vi "Grab -Main-CCD1 - 2.vi"(0 "Image in":T6(plugin-control)=refnum, 2 "right":dbl=1152.0, 3 "left":dbl=846.0, 5 "显示抓取图像":bool=TRUE, 7 "CCD2参数":T5={"Rectangle"={"Left"=1952, "Top"=146, "Right"=370, "Bottom"=2690, "Rotation"=45.0}, "Angle (degrees) "=90.0, "long"=150.0, "abgek"=-90.0, "Color"=16711680, "left threshold"=0.0, "Rectangle right"={"Left"=1952, "Top"=1596, "Right"=570, "Bottom"=2690, "Rotation"=45.0}, "long right"=150.0, "abgek right"=90.0, "Color 2"=16711680, "right threshold"=0.0, "left"=0.0, "right"=0.0, "Settings (Big)"={"Extraction Mode"=0, "Edge Threshold"=17, "Edge Filter Size"=1, "Min Length"=36, "Row Search Step Size"=13, "Col Search Step Size"=13, "Max Endpoint Gap"=10, "Closed"=FALSE, "Subpixel"=TRUE}, "Clamp Settings (Big)"={"Angle "=10.0, "Edge Polarity"={"Start"=0, "End"=0}}, " Settings top"={"Extraction Mode"=0, "Edge Threshold"=18, "Edge Filter Size"=1, "Min Length"=36, "Row Search Step Size"=64, "Col Search Step Size"=64, "Max Endpoint Gap"=10, "Closed"=FALSE, "Subpixel"=TRUE}, "Clamp Settings top "={"Angle "=10.0, "Edge Polarity"={"Start"=0, "End"=0}}, "Sub-Pixel Accuracy "=TRUE, "Threshold Parameters"={"Level Type"=enum."Absolute Value", "Threshold Level"=127, "Hysteresis"=2}, "Process "=enum."Get First + Last Edge", "Threshold Parameters 2"={"Level Type"=enum."Absolute Value", "Threshold Level"=127, "Hysteresis"=2}} {"Clamp Settings top"."Edge Polarity"."Start" items=["Any", "Rising", "Falling"]; "Clamp Settings top"."Edge Polarity"."End" items=["Any", "Rising", "Falling"]; "Settings top"."Extraction Mode" items=["Normal", "Uniform Regions"]; "Settings top"."Edge Filter Size" items=["Fine", "Normal", "Contour Tracing"]; "Settings top"."Max Endpoint Gap" min=0; "Settings top"."Col Search Step Size" min=1 max=255 step=1; "Settings top"."Row Search Step Size" min=1 max=255 step=1; "Settings top"."Min Length" min=0; "Settings top"."Edge Threshold" min=1 max=350 step=1; "Clamp Settings (Big)"."Edge Polarity"."Start" items=["Any", "Rising", "Falling"]; "Clamp Settings (Big)"."Edge Polarity"."End" items=["Any", "Rising", "Falling"]; "Settings (Big)"."Extraction Mode" items=["Normal", "Uniform Regions"]; "Settings (Big)"."Edge Filter Size" items=["Fine", "Normal", "Contour Tracing"]; "Settings (Big)"."Max Endpoint Gap" min=0; "Settings (Big)"."Col Search Step Size" min=1 max=255 step=1; "Settings (Big)"."Row Search Step Size" min=1 max=255 step=1; "Settings (Big)"."Min Length" min=0; "Settings (Big)"."Edge Threshold" min=1 max=350 step=1; "Rectangle right"."Rotation" format="%.2f"; "Rectangle right"."Left" scale=0.0..1024.0; "Rectangle right"."Right" scale=0.0..1024.0; "Rectangle"."Rotation" format="%.2f"; "Rectangle"."Left" scale=0.0..1024.0; "Rectangle"."Right" scale=0.0..1024.0}, 9 "ROI参数":T3={"Rectangle big CCD1"={"Left"=1952, "Top"=1596, "Right"=570, "Bottom"=2690, "Rotation"=45.0}, "Rectangle top CCD1 "={"Left"=1952, "Top"=1596, "Right"=570, "Bottom"=2690, "Rotation"=45.0}, "Line"={"Start X"=0, "Start Y"=0, "End X"=0, "End Y"=0}, "left line "=846.0, "right line"=1152.0} {"Line"."Start X" scale=0.0..1024.0; "Line"."End X" scale=0.0..1024.0; "Rectangle top CCD1"."Rotation" format="%.2f"; "Rectangle top CCD1"."Left" scale=0.0..1024.0; "Rectangle top CCD1"."Right" scale=0.0..1024.0; "Rectangle big CCD1"."Rotation" format="%.2f"; "Rectangle big CCD1"."Left" scale=0.0..1024.0; "Rectangle big CCD1"."Right" scale=0.0..1024.0}, 11 "error in (no error)":errorcluster caption="错误输入（无错误）") -> (4 "Image out":T6(plugin-control), 6 "NO LINES":bool, 8 "CCD2-L":bool, 10 "CCD2-R":bool, 15 "error out":errorcluster caption="错误输出")   [LabVIEW 2017]
doc: "The Grab VI acquires images continuously and displays the images in an image control using high-level acquisition VIs. A grab is appropriate for high-speed applications in which you need to process only one image at a time."
uses:
  <vilib>/vision/Pattern Matching.llb/IMAQ Curve Parameters.ctl
  Global System.vi
panel:
  out "下":dbl
  out "上":dbl
  in  "组合框":string(combo)="模式1"
  # "箭头指示参数"
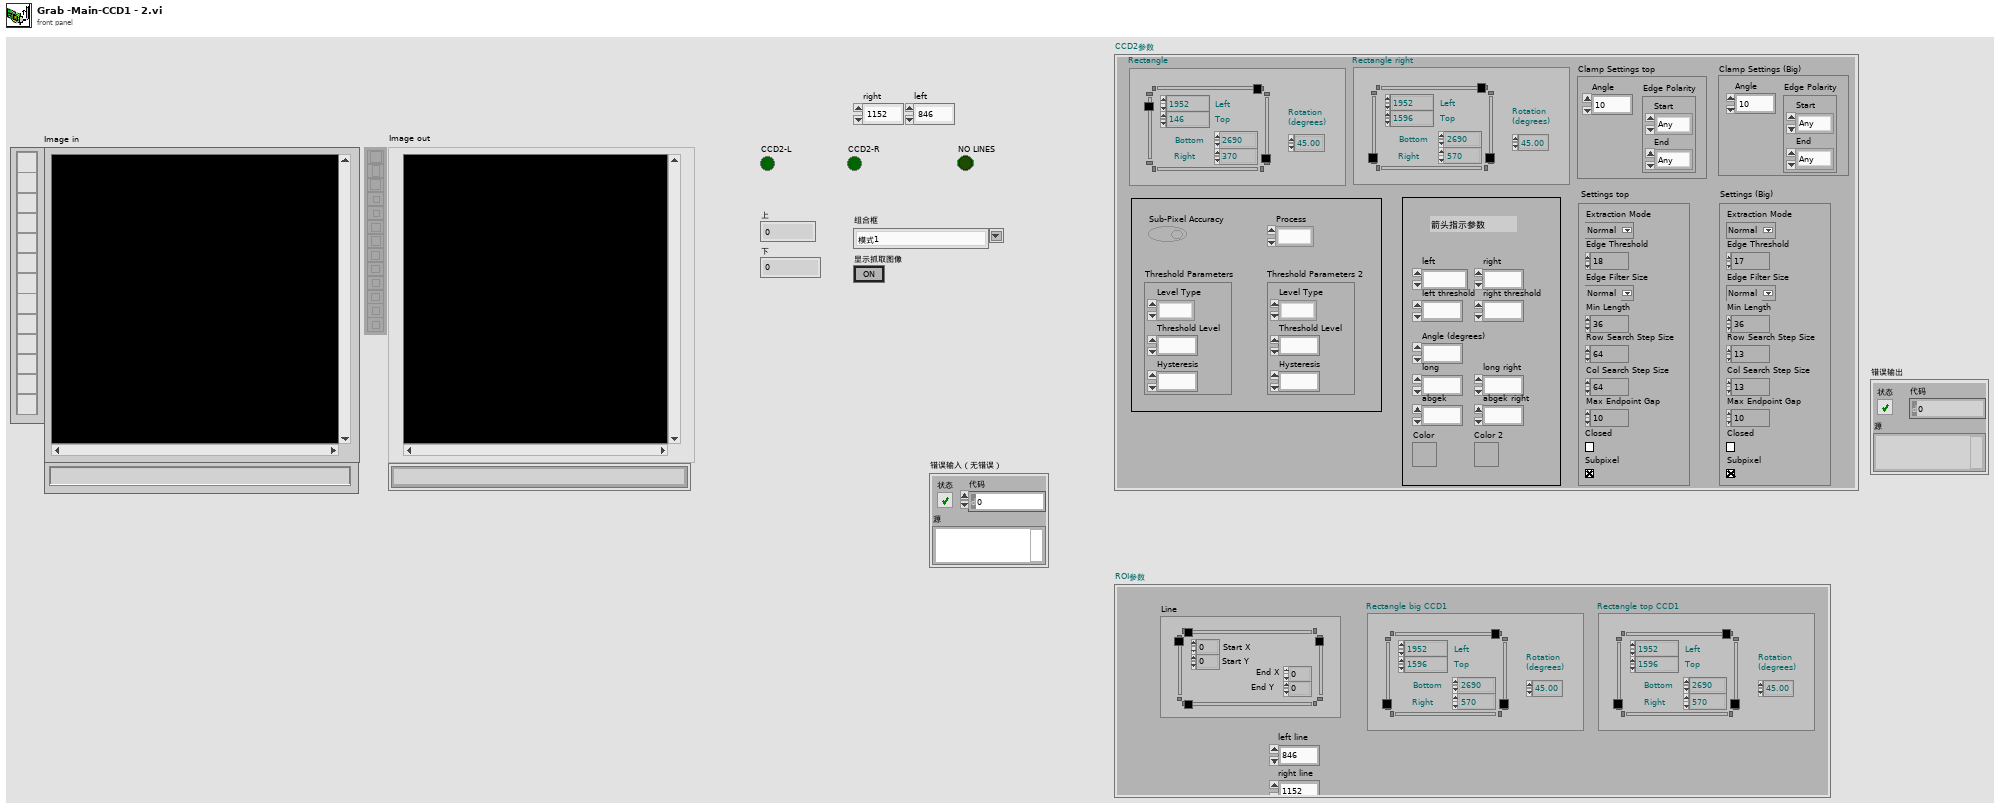
[diagram p1: front panel]
types:
  T1 = typedef "IMAQ Rectangle" = cluster{"Left":i32, "Top":i32, "Right":i32, "Bottom":i32, "Rotation":dbl}
  T2 = typedef "IMAQ Line" = cluster{"Start X":i32, "Start Y":i32, "End X":i32, "End Y":i32}
  T3 = cluster{"Rectangle big CCD1":T1, "Rectangle top CCD1 ":T1, "Line":T2, "left line ":dbl, "right line":dbl}
  T4 = typedef "IMAQ Curve Parameters.ctl" = cluster{"Extraction Mode":u32, "Edge Threshold":i32, "Edge Filter Size":u32, "Min Length":i32, "Row Search Step Size":i32, "Col Search Step Size":i32, "Max Endpoint Gap":i32, "Closed":bool, "Subpixel":bool}
  T5 = cluster{"Rectangle":T1, "Angle (degrees) ":sgl, "long":sgl, "abgek":dbl, "Color":u32, "left threshold":dbl, "Rectangle right":T1, "long right":sgl, "abgek right":dbl, "Color 2":u32, "right threshold":dbl, "left":dbl, "right":dbl, "Settings (Big)":T4, "Clamp Settings (Big)":cluster{"Angle ":dbl, "Edge Polarity":cluster{"Start":u32, "End":u32}}, " Settings top":T4, "Clamp Settings top ":cluster{"Angle ":dbl, "Edge Polarity":cluster{"Start":u32, "End":u32}}, "Sub-Pixel Accuracy ":bool, "Threshold Parameters":cluster{"Level Type":enum32{"Absolute Value", "Relative value"}, "Threshold Level":i32, "Hysteresis":i32}, "Process ":enum16{"Get First Edge", "Get First + Last Edge", "Get All Edges"}, "Threshold Parameters 2":cluster{"Level Type":enum32{"Absolute Value", "Relative value"}, "Threshold Level":i32, "Hysteresis":i32}}
  T6 = typedef "IMAQ Image.ctl" = refnum<image>
  T7 = cluster{"Clamp Points (Max Clamp 1)":cluster{"Pixels ":cluster{"Start":cluster{"X":dbl, "Y":dbl}, "End":cluster{"X":dbl, "Y":dbl}}, "Real World":cluster{"Start":cluster{"X":dbl, "Y":dbl}, "End":cluster{"X":dbl, "Y":dbl}}}, "Clamp Points (Max Clamp 2)":cluster{"Pixels ":cluster{"Start":cluster{"X":dbl, "Y":dbl}, "End":cluster{"X":dbl, "Y":dbl}}, "Real World":cluster{"Start":cluster{"X":dbl, "Y":dbl}, "End":cluster{"X":dbl, "Y":dbl}}}, "Clamp Points(top)":cluster{"Pixels ":cluster{"Start":cluster{"X":dbl, "Y":dbl}, "End":cluster{"X":dbl, "Y":dbl}}, "Real World":cluster{"Start":cluster{"X":dbl, "Y":dbl}, "End":cluster{"X":dbl, "Y":dbl}}}}
  T8 = cluster{"Angle ":dbl, "Edge Polarity":cluster{"Start":u32, "End":u32}}
  T9 = cluster{"Global Rectangle":i32[], "Contours":cluster{"ID":enum32{"External", "Internal"}, "Type":u32, "Coordinates":i32[]}[]}
  T10 = cluster{"Start":cluster{"X":dbl, "Y":dbl}, "End":cluster{"X":dbl, "Y":dbl}}
  T11 = cluster{"Pixels ":cluster{"Start":cluster{"X":dbl, "Y":dbl}, "End":cluster{"X":dbl, "Y":dbl}}, "Real World":cluster{"Start":cluster{"X":dbl, "Y":dbl}, "End":cluster{"X":dbl, "Y":dbl}}}
  T12 = cluster{"Left":i32, "Top":i32, "Right":i32, "Bottom":i32}
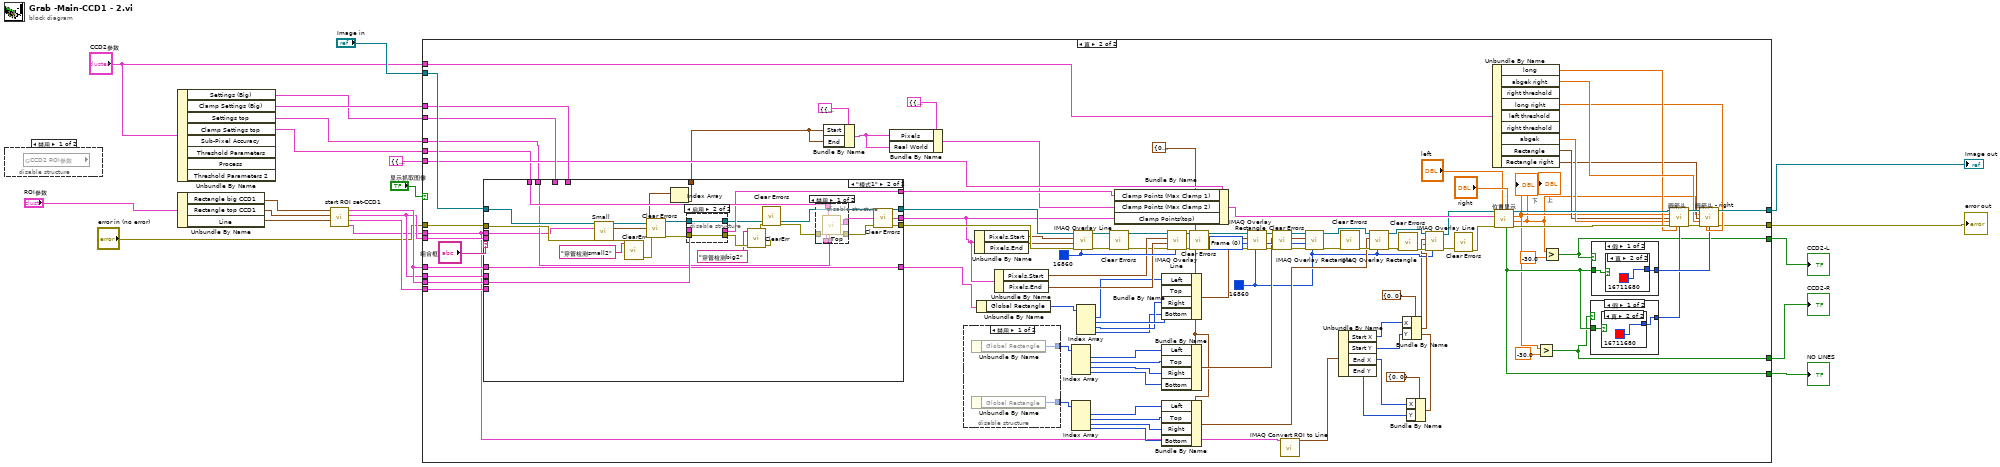
[diagram p0: block diagram]
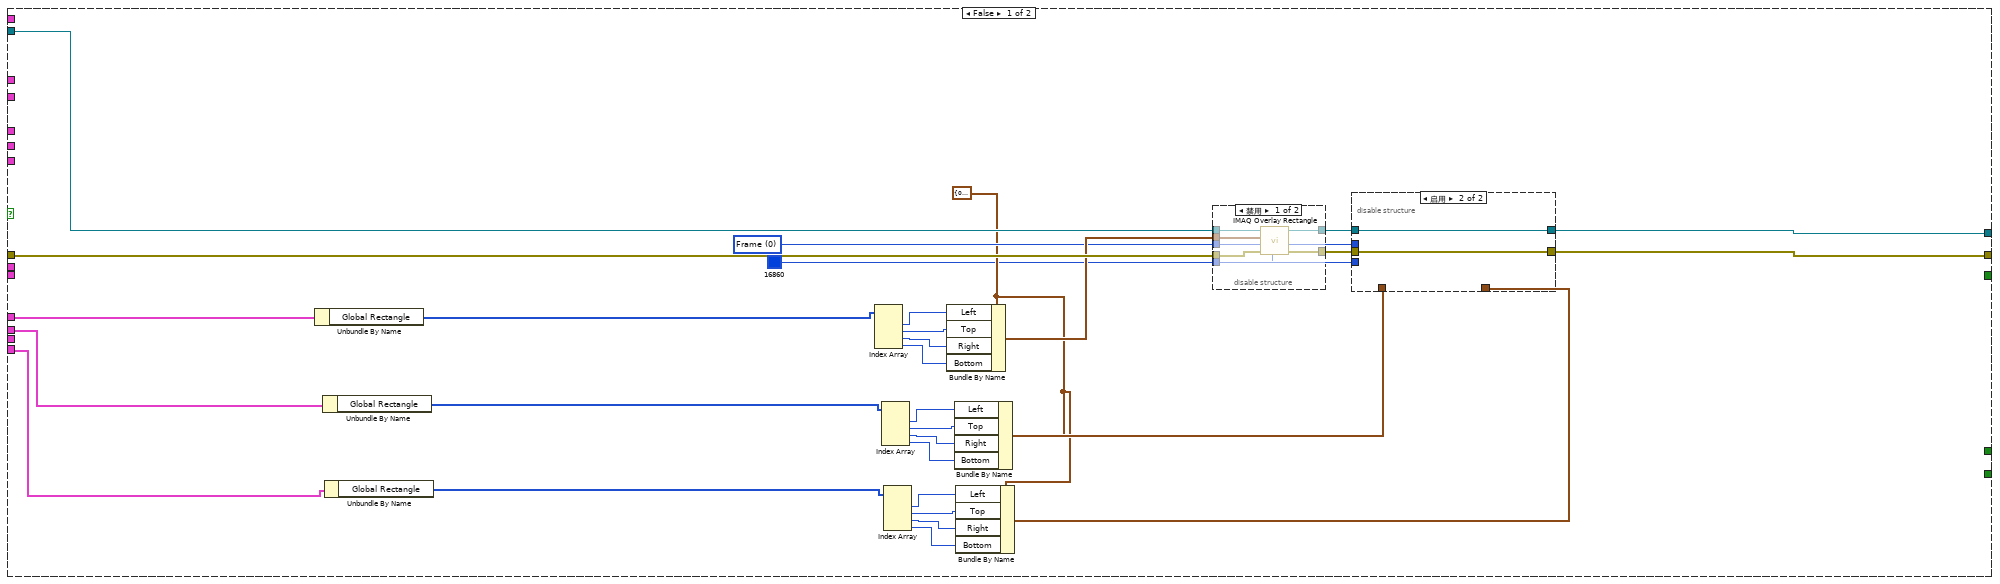
[diagram p3: hidden frame]
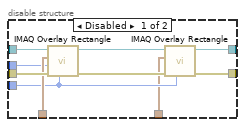
[diagram p5: hidden frame]
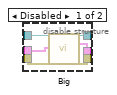
[diagram p8: hidden frame]
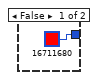
[diagram p10: hidden frame]
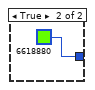
[diagram p11: hidden frame]
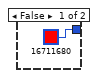
[diagram p12: hidden frame]
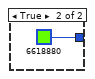
[diagram p13: hidden frame]
diagram:
  n1 = disable-structure shown="禁用" {
    frame Disabled {
      n2 = global read "Global System.vi" "CCD2 ROI参数"() -> ()  [unwired: 1 out]
    }
    frame Enabled {
    }
  }
  n3 = Unbundle By Name("CCD2参数") -> ("Settings (Big)"=w5:T4, "Clamp Settings (Big)"=w16:T8, "Settings top"=w12:T4, "Clamp Settings top"=w11:T8)  [unwired: 4 out]
  n4 = Unbundle By Name("ROI参数") -> ("Rectangle big CCD1"=w6:T1, "Rectangle top CCD1"=w7:T1, "Line"=w4:T2)
  n5 = call "start ROI set-CCD1.vi"("Rectangle big CCD1"=w6, "Line"=w4, "Rectangle top CCD1"=w7) -> ("ROI Descriptor (big)"=w15:T9, "ROI Descriptor (Small)"=w14:T9, "ROI Descriptor top"=w10:T9, "ROI Descriptor LINE"=w3:T9)  [unwired: 4 in]
  n6 = case shown="真" "显示抓取图像" {
    tunnel: [w27 w171] -> w17
    tunnel: "error in (no error)" -> [w39 w162]
    tunnel: [w26 w161] -> w2
    tunnel: w15 -> [w42 w134]
    tunnel: w14 -> [w41 w133]
    tunnel: "Image in" -> [w34 w128]
    tunnel: "CCD2参数" -> [_ w127]
    tunnel: [_ w75] -> w20
    tunnel: [_ w74] -> w19
    tunnel: [_ w126] -> w18
    tunnel: w16 -> [_ w125]
    tunnel: w5 -> [_ w124]
    tunnel: w15 -> [_ w123]
    tunnel: w14 -> [_ w122]
    tunnel: T7 {"Clamp Points (Max Clamp 1)"={"Pixels "={"Start"={"X"=889.781005859375, "Y"=1100.0}, "End"={"X"=1372.659423828125, "Y"=1100.0}}, "Real World"={"Start"={"X"=889.781005859375, "Y"=1100.0}, "End"={"X"=1372.659423828125, "Y"=1100.0}}}, "Clamp Points (Max Clamp 2)"={"Pixels "={"Start"={"X"=1112.3248291015625, "Y"=902.9254150390625}, "End"={"X"=1334.1685791015625, "Y"=893.0718994140625}}, "Real World"={"Start"={"X"=1112.3248291015625, "Y"=902.9254150390625}, "End"={"X"=1334.1685791015625, "Y"=893.0718994140625}}}, "Clamp Points(top)"={"Pixels "={"Start"={"X"=1112.3248291015625, "Y"=902.9254150390625}, "End"={"X"=1334.1685791015625, "Y"=893.0718994140625}}, "Real World"={"Start"={"X"=1112.3248291015625, "Y"=902.9254150390625}, "End"={"X"=1334.1685791015625, "Y"=893.0718994140625}}}} ("簇") -> [_ w116]
    tunnel: w12 -> [_ w115]
    tunnel: w11 -> [_ w114]
    tunnel: w10 -> [w23 w113]
    tunnel: w3 -> [_ w87]
    frame False {
      w25 = u32 16860 ("Color")
      w35 = u32 0 items=["Frame", "Fill", "Highlight"] ("Drawing Mode (Frame)")
      w28 = T12 {"Left"=0, "Top"=0, "Right"=0, "Bottom"=0} ("Rectangle")
      n7 = Unbundle By Name(w42) -> ("Global Rectangle"=w52:i32[])
      n8 = Unbundle By Name(w41) -> ("Global Rectangle"=w43:i32[])
      n9 = Unbundle By Name(w23) -> ("Global Rectangle"=w33:i32[])
      n10 = Index Array(array=w52) -> (element #1=w51:i32, element #2=w50:i32, element #3=w49:i32, element #4=w48:i32)  [unwired: 4 in]
      n11 = Index Array(array=w43) -> (element #1=w44:i32, element #2=w45:i32, element #3=w46:i32, element #4=w47:i32)  [unwired: 4 in]
      n12 = Index Array(array=w33) -> (element #1=w32:i32, element #2=w31:i32, element #3=w30:i32, element #4=w29:i32)  [unwired: 4 in]
      n13 = Bundle By Name(cluster=w28, "Left"=w51, "Top"=w50, "Right"=w49, "Bottom"=w48) -> (w37:T12)
      n14 = Bundle By Name(cluster=w28, "Left"=w44, "Top"=w45, "Right"=w46, "Bottom"=w47) -> (w36:T12)
      n15 = Bundle By Name(cluster=w28, "Left"=w32, "Top"=w31, "Right"=w30, "Bottom"=w29) -> (w24:T12)
      n16 = disable-structure shown="禁用" {
        disable-tunnel: [w59 _] -> w40
        disable-tunnel: w39 -> [w58 _]
        disable-tunnel: [w57 _] -> w38
        disable-tunnel: w37 -> [w56 _]
        disable-tunnel: w35 -> [w55 _]
        disable-tunnel: w34 -> [w54 _]
        disable-tunnel: w25 -> [w53 _]
        frame Disabled {
          n17 = call "IMAQ Overlay Rectangle"("Color"=w53, "error in (no error)"=w58, "Drawing Mode (Frame)"=w55, "Rectangle"=w56, "Image"=w54) -> ("error out"=w57:errorcluster, "Image Out"=w59:T6)  [unwired: 5 in]
        }
        frame Enabled {
        }
      }
      n18 = disable-structure shown="启用" {
        disable-tunnel: w40 -> [w69 w71]
        disable-tunnel: w38 -> [w68 w70]
        disable-tunnel: w36 -> [w67 _]
        disable-tunnel: w35 -> [w66 _]
        disable-tunnel: [w64 w71] -> w27
        disable-tunnel: [w63 w70] -> w26
        disable-tunnel: w25 -> [w61 _]
        disable-tunnel: w24 -> [w60 _]
        frame Disabled {
          n19 = call "IMAQ Overlay Rectangle"("Color"=w61, "error in (no error)"=w68, "Drawing Mode (Frame)"=w66, "Rectangle"=w67, "Image"=w69) -> ("error out"=w62:errorcluster, "Image Out"=w65:T6)  [unwired: 5 in]
          n20 = call "IMAQ Overlay Rectangle"("Color"=w61, "error in (no error)"=w62, "Rectangle"=w60, "Image"=w65) -> ("error out"=w63:errorcluster, "Image Out"=w64:T6)  [unwired: 6 in]
        }
        frame Enabled {
        }
      }
    }
    frame True {
      w137 = u32 0 items=["Frame", "Fill", "Highlight"] ("Drawing Mode (Frame)")
      w88 = u32 16860 ("Color")
      w153 = u32 16860 ("Color")
      w107 = T12 {"Left"=0, "Top"=0, "Right"=0, "Bottom"=0} ("Rectangle")
      n21 = case shown="\"模式1\"" "组合框" {
        tunnel: [w177 w184] -> w159
        tunnel: [w176 w194] -> w157
        tunnel: w128 -> [w177 w200]
        tunnel: w162 -> [w176 w199]
        tunnel: [_ w188] -> w149
        tunnel: w134 -> [_ w188]
        tunnel: w133 -> [_ _]
        tunnel: w125 -> [_ _]
        tunnel: w124 -> [_ _]
        tunnel: w123 -> [_ w193]
        tunnel: w122 -> [_ _]
        tunnel: w115 -> [_ w191]
        tunnel: w114 -> [_ w192]
        tunnel: w113 -> [_ _]
        tunnel: [_ w190] -> w96
        tunnel: [_ w189] -> w102
        tunnel: [_ w186] -> w98
        tunnel: w87 -> [_ w185]
        frame "假", Default {
        }
        frame "模式1" {
          n22 = call "Small"("Image In"=w200, "ROI Descriptor (Edge Detector 1)"=w185, "error in"=w199) -> ("Image Out"=w198:T6, "Edges Coordinates (Edge Detector 1)"=w187:cluster{"X":sgl, "Y":sgl}[], "error out"=w183:errorcluster)  [unwired: 20 in, 2 out]
          n23 = call "ClearErr.vi"("error in (no error)"=w183, "运行位置"="穿管检测small2") -> ("error out"=w182:errorcluster)  [unwired: 9 in]
          n24 = call <vilib>:"Clear Errors.vi"("error in (no error)"=w182) -> ("error out"=w196:errorcluster)  [unwired: 5 in, 1 out]
          n25 = Index Array(array=w187) -> (element=w186:cluster{"X":sgl, "Y":sgl})  [unwired: 1 in]
          n26 = disable-structure shown="启用" {
            disable-tunnel: w198 -> [w206 w208]
            disable-tunnel: w196 -> [w205 w207]
            disable-tunnel: w193 -> [w204 _]
            disable-tunnel: [w203 _] -> w189
            disable-tunnel: [w202 w208] -> w184
            disable-tunnel: [w201 w207] -> w181
            frame Disabled {
              n27 = call "Big"("Image In"=w206, "ROI Descriptor (Big)"=w204, "error in"=w205) -> ("Image Out"=w202:T6, "Clamp Points (Big)"=w203:T11, "error out"=w201:errorcluster)  [unwired: 22 in]
            }
            frame Enabled {
            }
          }
          n28 = call "ClearErr.vi"("error in (no error)"=w181, "运行位置"="穿管检测big2") -> ("error out"=w180:errorcluster)  [unwired: 9 in]
          n29 = call <vilib>:"Clear Errors.vi"("error in (no error)"=w180) -> ("error out"=w195:errorcluster)  [unwired: 5 in, 1 out]
          n30 = disable-structure shown="禁用" {
            disable-tunnel: [w214 _] -> w197
            disable-tunnel: w195 -> [w213 _]
            disable-tunnel: w192 -> [w212 _]
            disable-tunnel: w191 -> [w211 _]
            disable-tunnel: [w210 _] -> w190
            disable-tunnel: _ -> [w209 _]
            frame Disabled {
              n31 = call "Top"("error in"=w213, "ROI Descriptor (top)"=w209, "Clamp Settings (top)"=w212, "Curve Extraction Settings (top)"=w211) -> ("Clamp Points (top)"=w210:T11, "error out"=w214:errorcluster)  [unwired: 21 in, 1 out]
            }
            frame Enabled {
            }
          }
          n32 = call <vilib>:"Clear Errors.vi"("error in (no error)"=w197) -> ("error out"=w194:errorcluster)  [unwired: 5 in, 1 out]
        }
      }
      n33 = Bundle By Name(cluster=T10 {"Start"={"X"=0.0, "Y"=0.0}, "End"={"X"=0.0, "Y"=0.0}} ("Pixels"), "Start"=w98, "End"=w98) -> (w97:T10)
      n34 = Bundle By Name(cluster=T11 {"Pixels "={"Start"={"X"=0.0, "Y"=0.0}, "End"={"X"=0.0, "Y"=0.0}}, "Real World"={"Start"={"X"=0.0, "Y"=0.0}, "End"={"X"=0.0, "Y"=0.0}}} ("Clamp Points (Max Clamp 2)"), "Pixels"=w97, "Real World"=w97) -> (w100:T11)
      n35 = disable-structure shown="禁用" {
        disable-tunnel: [w175 _] -> w138
        disable-tunnel: [w174 _] -> w112
        frame Disabled {
          n36 = Unbundle By Name() -> ("Global Rectangle"=w175:i32[])  [unwired: 1 in]
          n37 = Unbundle By Name() -> ("Global Rectangle"=w174:i32[])  [unwired: 1 in]
        }
        frame Enabled {
        }
      }
      n38 = Unbundle By Name(w96) -> ("Pixels.Start"=w155:cluster{"X":dbl, "Y":dbl}, "Pixels.End"=w154:cluster{"X":dbl, "Y":dbl})
      n39 = Unbundle By Name(w149) -> ("Global Rectangle"=w148:i32[])
      n40 = Unbundle By Name(w96) -> ("Pixels.Start"=w152:cluster{"X":dbl, "Y":dbl}, "Pixels.End"=w151:cluster{"X":dbl, "Y":dbl})
      n41 = Index Array(array=w138) -> (element #1=w139:i32, element #2=w140:i32, element #3=w141:i32, element #4=w142:i32)  [unwired: 4 in]
      n42 = Index Array(array=w112) -> (element #1=w111:i32, element #2=w110:i32, element #3=w109:i32, element #4=w108:i32)  [unwired: 4 in]
      n43 = call "IMAQ Overlay Line"("Color"=w153, "error in (no error)"=w157, "End Point"=w154, "Start Point"=w155, "Image"=w159) -> ("error out"=w156:errorcluster, "Image Out"=w158:T6)  [unwired: 5 in]
      n44 = Index Array(array=w148) -> (element #1=w147:i32, element #2=w146:i32, element #3=w145:i32, element #4=w144:i32)  [unwired: 4 in]
      n45 = call <vilib>:"Clear Errors.vi"("error in (no error)"=w156) -> ("error out"=w132:errorcluster)  [unwired: 5 in, 1 out]
      n46 = Bundle By Name(cluster=w116, "Clamp Points (Max Clamp 1)"=w102, "Clamp Points (Max Clamp 2)"=w100, "Clamp Points(top)"=w96) -> (w117:T7)
      n47 = Bundle By Name(cluster=w107, "Left"=w147, "Top"=w146, "Right"=w145, "Bottom"=w144) -> (w143:T12)
      n48 = Bundle By Name(cluster=w107, "Left"=w139, "Top"=w140, "Right"=w141, "Bottom"=w142) -> (w135:T12)
      n49 = Bundle By Name(cluster=w107, "Left"=w111, "Top"=w110, "Right"=w109, "Bottom"=w108) -> (w103:T12)
      n50 = call "IMAQ Overlay Line"("Color"=w153, "error in (no error)"=w132, "End Point"=w151, "Start Point"=w152, "Image"=w158) -> ("error out"=w78:errorcluster, "Image Out"=w79:T6)  [unwired: 5 in]
      n51 = call <vilib>:"Clear Errors.vi"("error in (no error)"=w78) -> ("error out"=w77:errorcluster)  [unwired: 5 in, 1 out]
      n52 = call "IMAQ Overlay Rectangle"("Color"=w88, "error in (no error)"=w77, "Drawing Mode (Frame)"=w137, "Rectangle"=w143, "Image"=w79) -> ("error out"=w76:errorcluster, "Image Out"=w150:T6)  [unwired: 5 in]
      n53 = call <vilib>:"Clear Errors.vi"("error in (no error)"=w76) -> ("error out"=w131:errorcluster)  [unwired: 5 in, 1 out]
      n54 = call "IMAQ Convert ROI to Line"("ROI Descriptor"=w87) -> ("Line"=w86:T2)  [unwired: 8 in, 1 out]
      n55 = call "IMAQ Overlay Rectangle"("Color"=w88, "error in (no error)"=w131, "Drawing Mode (Frame)"=w137, "Rectangle"=w135, "Image"=w150) -> ("error out"=w136:errorcluster, "Image Out"=w104:T6)  [unwired: 5 in]
      n56 = Unbundle By Name(w86) -> ("Start X"=w85:i32, "Start Y"=w84:i32, "End X"=w81:i32, "End Y"=w80:i32)
      n57 = call <vilib>:"Clear Errors.vi"("error in (no error)"=w136) -> ("error out"=w105:errorcluster)  [unwired: 5 in, 1 out]
      n58 = call "IMAQ Overlay Rectangle"("Color"=w88, "error in (no error)"=w105, "Rectangle"=w103, "Image"=w104) -> ("error out"=w106:errorcluster, "Image Out"=w92:T6)  [unwired: 6 in]
      n59 = call <vilib>:"Clear Errors.vi"("error in (no error)"=w106) -> ("error out"=w95:errorcluster)  [unwired: 5 in, 1 out]
      n60 = Bundle By Name(cluster=cluster{"X":i32, "Y":i32} {"X"=0, "Y"=0} ("Start Point"), "X"=w85, "Y"=w84) -> (w89:cluster{"X":i32, "Y":i32})
      n61 = Bundle By Name(cluster=cluster{"X":i32, "Y":i32} {"X"=0, "Y"=0} ("Start Point"), "X"=w81, "Y"=w80) -> (w82:cluster{"X":i32, "Y":i32})
      n62 = call "IMAQ Overlay Line"("Color"=w88, "error in (no error)"=w95, "End Point"=w82, "Start Point"=w89, "Image"=w92) -> ("error out"=w94:errorcluster, "Image Out"=w91:T6)  [unwired: 5 in]
      n63 = call <vilib>:"Clear Errors.vi"("error in (no error)"=w94) -> ("error out"=w93:errorcluster)  [unwired: 5 in, 1 out]
      n64 = Unbundle By Name(w127) -> ("long"=w167:sgl, "abgek right"=w170:dbl, "long right"=w166:sgl, "abgek"=w165:dbl, "Rectangle"=w164:T1, "Rectangle right"=w163:T1)  [unwired: 3 out]
      n65 = call "位置显示.vi"("right"="right", "left"="left", "error in (no error) 2"=w93, "簇"=w117, "Image in"=w91) -> ("error out"=w169:errorcluster, "左"=w118:dbl, "右"=w119:dbl, "Image out"=w173:T6, "x或y？"=w126:bool)  [unwired: 2 in]
      "上" <- w119
      "下" <- w118
      n66 = Greater?(x=w119, y=-30.0) -> (0:w74:bool)
      n67 = Greater?(x=w118, y=-30.0) -> (0:w75:bool)
      n68 = case shown="假" w74 {
        tunnel: [w221 u32 6618880 ("Color")] -> w120
        tunnel: w126 -> [w220 _]
        frame False {
          n69 = case shown="真" w220 {
            tunnel: [u32 16711680 ("Color") u32 16711680 ("Color")] -> w221
            frame False {
            }
            frame True {
            }
          }
        }
        frame True {
        }
      }
      n70 = case shown="假" w75 {
        tunnel: [w216 u32 6618880 ("Color")] -> w121
        tunnel: w126 -> [w215 _]
        frame False {
          n71 = case shown="真" w215 {
            tunnel: [u32 16711680 ("Color") u32 16711680 ("Color")] -> w216
            frame False {
            }
            frame True {
            }
          }
        }
        frame True {
        }
      }
      n72 = call "画箭头.vi"("Image 2"=w173, "距离"=w119, "Rectangle"=w164, "abgek"=w165, "error in (no error)"=w169, "long"=w167, "Color 2"=w120) -> ("Image"=w172:T6, "error out"=w168:errorcluster)  [unwired: 7 in]
      n73 = call "画箭头 - right.vi"("Image 2"=w172, "距离"=w118, "Rectangle"=w163, "abgek"=w170, "error in (no error)"=w168, "long"=w166, "Color 2"=w121) -> ("Image out"=w171:T6, "error out"=w161:errorcluster)  [unwired: 7 in]
    }
  }
  "error out" <- w2
  "CCD2-L" <- w20
  "CCD2-R" <- w19
  "NO LINES" <- w18
  "Image out" <- w17
